vi "Dresden R2R Sputter 03.02.2018 IY24.vi"() -> ()   [LabVIEW 2009] (continued)
                    n2885 = stacked-sequence {
                      frame #0 {
                        n2886 = local write "Pps_code_entry"("PF174=" ("Pps_code_entry")) -> ()
                      }
                      frame #1 {
                        n2887 = Wait (ms)(milliseconds to wait=u32 500) -> ()  [unwired: 1 out]
                      }
                      frame #2 {
                        n2888 = local write "Ppsok"(TRUE ("Ppsok")) -> ()
                      }
                    }
                  }
                  frame #1 {
                    n2889 = stacked-sequence {
                      frame #0 {
                        n2890 = local write "Pps_code_entry"("PF173=" ("Pps_code_entry")) -> ()
                      }
                      frame #1 {
                        n2891 = Wait (ms)(milliseconds to wait=u32 500) -> ()  [unwired: 1 out]
                      }
                      frame #2 {
                        n2892 = local write "Ppsok"(TRUE ("Ppsok")) -> ()
                      }
                    }
                  }
                }
              }
            }
            n2893 = case shown="True" w4809 {
              tunnel: w4813 -> [_ w5102]
              frame #0 {
              }
              frame #1 {
                n2894 = case shown="False" w5102 {
                  frame #0 {
                    n2895 = stacked-sequence {
                      frame #0 {
                        n2896 = local write "Pps_code_entry"("PF206=" ("Pps_code_entry")) -> ()
                      }
                      frame #1 {
                        n2897 = Wait (ms)(milliseconds to wait=u32 500) -> ()  [unwired: 1 out]
                      }
                      frame #2 {
                        n2898 = local write "Ppsok"(TRUE ("Ppsok")) -> ()
                      }
                    }
                  }
                  frame #1 {
                    n2899 = stacked-sequence {
                      frame #0 {
                        n2900 = local write "Pps_code_entry"("PF205=" ("Pps_code_entry")) -> ()
                      }
                      frame #1 {
                        n2901 = Wait (ms)(milliseconds to wait=u32 500) -> ()  [unwired: 1 out]
                      }
                      frame #2 {
                        n2902 = local write "Ppsok"(TRUE ("Ppsok")) -> ()
                      }
                    }
                  }
                }
              }
            }
            n2903 = case shown="True" w4969 {
              tunnel: w4973 -> [_ w5333]
              frame #0 {
              }
              frame #1 {
                n2904 = case shown="False" w5333 {
                  frame #0 {
                    n2905 = stacked-sequence {
                      frame #0 {
                        n2906 = local write "Pps_code_entry"("PF138=" ("Pps_code_entry")) -> ()
                      }
                      frame #1 {
                        n2907 = Wait (ms)(milliseconds to wait=u32 500) -> ()  [unwired: 1 out]
                      }
                      frame #2 {
                        n2908 = local write "Ppsok"(TRUE ("Ppsok")) -> ()
                      }
                    }
                  }
                  frame #1 {
                    n2909 = stacked-sequence {
                      frame #0 {
                        n2910 = local write "Pps_code_entry"("PF137=" ("Pps_code_entry")) -> ()
                      }
                      frame #1 {
                        n2911 = Wait (ms)(milliseconds to wait=u32 500) -> ()  [unwired: 1 out]
                      }
                      frame #2 {
                        n2912 = local write "Ppsok"(TRUE ("Ppsok")) -> ()
                      }
                    }
                  }
                }
              }
            }
            n2913 = case shown="True" w4828 {
              tunnel: w4824 -> [_ w5081]
              frame #0 {
              }
              frame #1 {
                n2914 = case shown="False" w5081 {
                  frame #0 {
                    n2915 = stacked-sequence {
                      frame #0 {
                        n2916 = local write "Pps_code_entry"("PF208=" ("Pps_code_entry")) -> ()
                      }
                      frame #1 {
                        n2917 = Wait (ms)(milliseconds to wait=u32 500) -> ()  [unwired: 1 out]
                      }
                      frame #2 {
                        n2918 = local write "Ppsok"(TRUE ("Ppsok")) -> ()
                      }
                    }
                  }
                  frame #1 {
                    n2919 = stacked-sequence {
                      frame #0 {
                        n2920 = local write "Pps_code_entry"("PF207=" ("Pps_code_entry")) -> ()
                      }
                      frame #1 {
                        n2921 = Wait (ms)(milliseconds to wait=u32 500) -> ()  [unwired: 1 out]
                      }
                      frame #2 {
                        n2922 = local write "Ppsok"(TRUE ("Ppsok")) -> ()
                      }
                    }
                  }
                }
              }
            }
            n2923 = case shown="True" w4988 {
              tunnel: w4984 -> [_ w5312]
              frame #0 {
              }
              frame #1 {
                n2924 = case shown="False" w5312 {
                  frame #0 {
                    n2925 = stacked-sequence {
                      frame #0 {
                        n2926 = local write "Pps_code_entry"("PF140=" ("Pps_code_entry")) -> ()
                      }
                      frame #1 {
                        n2927 = Wait (ms)(milliseconds to wait=u32 500) -> ()  [unwired: 1 out]
                      }
                      frame #2 {
                        n2928 = local write "Ppsok"(TRUE ("Ppsok")) -> ()
                      }
                    }
                  }
                  frame #1 {
                    n2929 = stacked-sequence {
                      frame #0 {
                        n2930 = local write "Pps_code_entry"("PF139=" ("Pps_code_entry")) -> ()
                      }
                      frame #1 {
                        n2931 = Wait (ms)(milliseconds to wait=u32 500) -> ()  [unwired: 1 out]
                      }
                      frame #2 {
                        n2932 = local write "Ppsok"(TRUE ("Ppsok")) -> ()
                      }
                    }
                  }
                }
              }
            }
            n2933 = case shown="True" w4869 {
              tunnel: w4873 -> [_ w5235]
              frame #0 {
              }
              frame #1 {
                n2934 = case shown="False" w5235 {
                  frame #0 {
                    n2935 = stacked-sequence {
                      frame #0 {
                        n2936 = local write "Pps_code_entry"("PF170=" ("Pps_code_entry")) -> ()
                      }
                      frame #1 {
                        n2937 = Wait (ms)(milliseconds to wait=u32 500) -> ()  [unwired: 1 out]
                      }
                      frame #2 {
                        n2938 = local write "Ppsok"(TRUE ("Ppsok")) -> ()
                      }
                    }
                  }
                  frame #1 {
                    n2939 = stacked-sequence {
                      frame #0 {
                        n2940 = local write "Pps_code_entry"("PF169=" ("Pps_code_entry")) -> ()
                      }
                      frame #1 {
                        n2941 = Wait (ms)(milliseconds to wait=u32 500) -> ()  [unwired: 1 out]
                      }
                      frame #2 {
                        n2942 = local write "Ppsok"(TRUE ("Ppsok")) -> ()
                      }
                    }
                  }
                }
              }
            }
            n2943 = case shown="True" w4904 {
              tunnel: w4908 -> [_ w5179]
              frame #0 {
              }
              frame #1 {
                n2944 = case shown="False" w5179 {
                  frame #0 {
                    n2945 = stacked-sequence {
                      frame #0 {
                        n2946 = local write "Pps_code_entry"("PF184=" ("Pps_code_entry")) -> ()
                      }
                      frame #1 {
                        n2947 = Wait (ms)(milliseconds to wait=u32 500) -> ()  [unwired: 1 out]
                      }
                      frame #2 {
                        n2948 = local write "Ppsok"(TRUE ("Ppsok")) -> ()
                      }
                    }
                  }
                  frame #1 {
                    n2949 = stacked-sequence {
                      frame #0 {
                        n2950 = local write "Pps_code_entry"("PF183=" ("Pps_code_entry")) -> ()
                      }
                      frame #1 {
                        n2951 = Wait (ms)(milliseconds to wait=u32 500) -> ()  [unwired: 1 out]
                      }
                      frame #2 {
                        n2952 = local write "Ppsok"(TRUE ("Ppsok")) -> ()
                      }
                    }
                  }
                }
              }
            }
            n2953 = case shown="True" w4798 {
              tunnel: w4794 -> [_ w5123]
              frame #0 {
              }
              frame #1 {
                n2954 = case shown="True" w5123 {
                  frame #0 {
                    n2955 = stacked-sequence {
                      frame #0 {
                        n2956 = local write "Pps_code_entry"("PF204=" ("Pps_code_entry")) -> ()
                      }
                      frame #1 {
                        n2957 = Wait (ms)(milliseconds to wait=u32 500) -> ()  [unwired: 1 out]
                      }
                      frame #2 {
                        n2958 = local write "Ppsok"(TRUE ("Ppsok")) -> ()
                      }
                    }
                  }
                  frame #1 {
                    n2959 = stacked-sequence {
                      frame #0 {
                        n2960 = local write "Pps_code_entry"("PF203=" ("Pps_code_entry")) -> ()
                      }
                      frame #1 {
                        n2961 = Wait (ms)(milliseconds to wait=u32 500) -> ()  [unwired: 1 out]
                      }
                      frame #2 {
                        n2962 = local write "Ppsok"(TRUE ("Ppsok")) -> ()
                      }
                    }
                  }
                }
              }
            }
            n2963 = case shown="True" w5028 {
              tunnel: w5024 -> [_ w5438]
              frame #0 {
              }
              frame #1 {
                n2964 = case shown="True" w5438 {
                  frame #0 {
                    n2965 = stacked-sequence {
                      frame #0 {
                        n2966 = local write "Pps_code_entry"("PF108=" ("Pps_code_entry")) -> ()
                      }
                      frame #1 {
                        n2967 = Wait (ms)(milliseconds to wait=u32 500) -> ()  [unwired: 1 out]
                      }
                      frame #2 {
                        n2968 = local write "Ppsok"(TRUE ("Ppsok")) -> ()
                      }
                    }
                  }
                  frame #1 {
                    n2969 = stacked-sequence {
                      frame #0 {
                        n2970 = local write "Pps_code_entry"("PF107=" ("Pps_code_entry")) -> ()
                      }
                      frame #1 {
                        n2971 = Wait (ms)(milliseconds to wait=u32 500) -> ()  [unwired: 1 out]
                      }
                      frame #2 {
                        n2972 = local write "Ppsok"(TRUE ("Ppsok")) -> ()
                      }
                    }
                  }
                }
              }
            }
            n2973 = case shown="True" w4958 {
              tunnel: w4954 -> [_ w5354]
              frame #0 {
              }
              frame #1 {
                n2974 = case shown="True" w5354 {
                  frame #0 {
                    n2975 = stacked-sequence {
                      frame #0 {
                        n2976 = local write "Pps_code_entry"("PF136=" ("Pps_code_entry")) -> ()
                      }
                      frame #1 {
                        n2977 = Wait (ms)(milliseconds to wait=u32 500) -> ()  [unwired: 1 out]
                      }
                      frame #2 {
                        n2978 = local write "Ppsok"(TRUE ("Ppsok")) -> ()
                      }
                    }
                  }
                  frame #1 {
                    n2979 = stacked-sequence {
                      frame #0 {
                        n2980 = local write "Pps_code_entry"("PF135=" ("Pps_code_entry")) -> ()
                      }
                      frame #1 {
                        n2981 = Wait (ms)(milliseconds to wait=u32 500) -> ()  [unwired: 1 out]
                      }
                      frame #2 {
                        n2982 = local write "Ppsok"(TRUE ("Ppsok")) -> ()
                      }
                    }
                  }
                }
              }
            }
            n2983 = case shown="True" w4923 {
              tunnel: w4919 -> [_ w5291]
              frame #0 {
              }
              frame #1 {
                n2984 = case shown="True" w5291 {
                  frame #0 {
                    n2985 = stacked-sequence {
                      frame #0 {
                        n2986 = local write "Pps_code_entry"("PF150=" ("Pps_code_entry")) -> ()
                      }
                      frame #1 {
                        n2987 = Wait (ms)(milliseconds to wait=u32 500) -> ()  [unwired: 1 out]
                      }
                      frame #2 {
                        n2988 = local write "Ppsok"(TRUE ("Ppsok")) -> ()
                      }
                    }
                  }
                  frame #1 {
                    n2989 = stacked-sequence {
                      frame #0 {
                        n2990 = local write "Pps_code_entry"("PF149=" ("Pps_code_entry")) -> ()
                      }
                      frame #1 {
                        n2991 = Wait (ms)(milliseconds to wait=u32 500) -> ()  [unwired: 1 out]
                      }
                      frame #2 {
                        n2992 = local write "Ppsok"(TRUE ("Ppsok")) -> ()
                      }
                    }
                  }
                }
              }
            }
            n2993 = case shown="True" w5009 {
              tunnel: w5013 -> [_ w5417]
              frame #0 {
              }
              frame #1 {
                n2994 = case shown="False" w5417 {
                  frame #0 {
                    n2995 = stacked-sequence {
                      frame #0 {
                        n2996 = local write "Pps_code_entry"("PF110=" ("Pps_code_entry")) -> ()
                      }
                      frame #1 {
                        n2997 = Wait (ms)(milliseconds to wait=u32 500) -> ()  [unwired: 1 out]
                      }
                      frame #2 {
                        n2998 = local write "Ppsok"(TRUE ("Ppsok")) -> ()
                      }
                    }
                  }
                  frame #1 {
                    n2999 = stacked-sequence {
                      frame #0 {
                        n3000 = local write "Pps_code_entry"("PF109=" ("Pps_code_entry")) -> ()
                      }
                      frame #1 {
                        n3001 = Wait (ms)(milliseconds to wait=u32 500) -> ()  [unwired: 1 out]
                      }
                      frame #2 {
                        n3002 = local write "Ppsok"(TRUE ("Ppsok")) -> ()
                      }
                    }
                  }
                }
              }
            }
            n3003 = case shown="True" w4900 {
              tunnel: w4899 -> [_ w5277]
              frame #0 {
              }
              frame #1 {
                n3004 = case shown="False" w5277 {
                  frame #0 {
                    n3005 = stacked-sequence {
                      frame #0 {
                        n3006 = local write "Pps_code_entry"("PF166=" ("Pps_code_entry")) -> ()
                      }
                      frame #1 {
                        n3007 = Wait (ms)(milliseconds to wait=u32 500) -> ()  [unwired: 1 out]
                      }
                      frame #2 {
                        n3008 = local write "Ppsok"(TRUE ("Ppsok")) -> ()
                      }
                    }
                  }
                  frame #1 {
                    n3009 = stacked-sequence {
                      frame #0 {
                        n3010 = local write "Pps_code_entry"("PF165=" ("Pps_code_entry")) -> ()
                      }
                      frame #1 {
                        n3011 = Wait (ms)(milliseconds to wait=u32 500) -> ()  [unwired: 1 out]
                      }
                      frame #2 {
                        n3012 = local write "Ppsok"(TRUE ("Ppsok")) -> ()
                      }
                    }
                  }
                }
              }
            }
            n3013 = case shown="True" w4898 {
              tunnel: w4894 -> [_ w5270]
              frame #0 {
              }
              frame #1 {
                n3014 = case shown="False" w5270 {
                  frame #0 {
                    n3015 = stacked-sequence {
                      frame #0 {
                        n3016 = local write "Pps_code_entry"("PF168=" ("Pps_code_entry")) -> ()
                      }
                      frame #1 {
                        n3017 = Wait (ms)(milliseconds to wait=u32 500) -> ()  [unwired: 1 out]
                      }
                      frame #2 {
                        n3018 = local write "Ppsok"(TRUE ("Ppsok")) -> ()
                      }
                    }
                  }
                  frame #1 {
                    n3019 = stacked-sequence {
                      frame #0 {
                        n3020 = local write "Pps_code_entry"("PF167=" ("Pps_code_entry")) -> ()
                      }
                      frame #1 {
                        n3021 = Wait (ms)(milliseconds to wait=u32 500) -> ()  [unwired: 1 out]
                      }
                      frame #2 {
                        n3022 = local write "Ppsok"(TRUE ("Ppsok")) -> ()
                      }
                    }
                  }
                }
              }
            }
            n3023 = case shown="True" w5039 {
              tunnel: w5043 -> [_ w5459]
              frame #0 {
              }
              frame #1 {
                n3024 = case shown="False" w5459 {
                  frame #0 {
                    n3025 = stacked-sequence {
                      frame #0 {
                        n3026 = local write "Pps_code_entry"("PF106=" ("Pps_code_entry")) -> ()
                      }
                      frame #1 {
                        n3027 = Wait (ms)(milliseconds to wait=u32 500) -> ()  [unwired: 1 out]
                      }
                      frame #2 {
                        n3028 = local write "Ppsok"(TRUE ("Ppsok")) -> ()
                      }
                    }
                  }
                  frame #1 {
                    n3029 = stacked-sequence {
                      frame #0 {
                        n3030 = local write "Pps_code_entry"("PF105=" ("Pps_code_entry")) -> ()
                      }
                      frame #1 {
                        n3031 = Wait (ms)(milliseconds to wait=u32 500) -> ()  [unwired: 1 out]
                      }
                      frame #2 {
                        n3032 = local write "Ppsok"(TRUE ("Ppsok")) -> ()
                      }
                    }
                  }
                }
              }
            }
            n3033 = case shown="True" w4767 {
              tunnel: w4768 -> [_ w5165]
              frame #0 {
              }
              frame #1 {
                n3034 = case shown="True" w5165 {
                  frame #0 {
                    n3035 = stacked-sequence {
                      frame #0 {
                        n3036 = local write "Pps_code_entry"("PF200=" ("Pps_code_entry")) -> ()
                      }
                      frame #1 {
                        n3037 = Wait (ms)(milliseconds to wait=u32 500) -> ()  [unwired: 1 out]
                      }
                      frame #2 {
                        n3038 = local write "Ppsok"(TRUE ("Ppsok")) -> ()
                      }
                    }
                  }
                  frame #1 {
                    n3039 = stacked-sequence {
                      frame #0 {
                        n3040 = local write "Pps_code_entry"("PF199=" ("Pps_code_entry")) -> ()
                      }
                      frame #1 {
                        n3041 = Wait (ms)(milliseconds to wait=u32 500) -> ()  [unwired: 1 out]
                      }
                      frame #2 {
                        n3042 = local write "Ppsok"(TRUE ("Ppsok")) -> ()
                      }
                    }
                  }
                }
              }
            }
            n3043 = case shown="True" w4769 {
              tunnel: w4773 -> [_ w5158]
              frame #0 {
              }
              frame #1 {
                n3044 = case shown="True" w5158 {
                  frame #0 {
                    n3045 = stacked-sequence {
                      frame #0 {
                        n3046 = local write "Pps_code_entry"("PF202=" ("Pps_code_entry")) -> ()
                      }
                      frame #1 {
                        n3047 = Wait (ms)(milliseconds to wait=u32 500) -> ()  [unwired: 1 out]
                      }
                      frame #2 {
                        n3048 = local write "Ppsok"(TRUE ("Ppsok")) -> ()
                      }
                    }
                  }
                  frame #1 {
                    n3049 = stacked-sequence {
                      frame #0 {
                        n3050 = local write "Pps_code_entry"("PF201=" ("Pps_code_entry")) -> ()
                      }
                      frame #1 {
                        n3051 = Wait (ms)(milliseconds to wait=u32 500) -> ()  [unwired: 1 out]
                      }
                      frame #2 {
                        n3052 = local write "Ppsok"(TRUE ("Ppsok")) -> ()
                      }
                    }
                  }
                }
              }
            }
            n3053 = case shown="True" w4927 {
              tunnel: w4928 -> [_ w5396]
              frame #0 {
              }
              frame #1 {
                n3054 = case shown="False" w5396 {
                  frame #0 {
                    n3055 = stacked-sequence {
                      frame #0 {
                        n3056 = local write "Pps_code_entry"("PF133=" ("Pps_code_entry")) -> ()
                      }
                      frame #1 {
                        n3057 = Wait (ms)(milliseconds to wait=u32 500) -> ()  [unwired: 1 out]
                      }
                      frame #2 {
                        n3058 = local write "Ppsok"(TRUE ("Ppsok")) -> ()
                      }
                    }
                  }
                  frame #1 {
                    n3059 = stacked-sequence {
                      frame #0 {
                        n3060 = local write "Pps_code_entry"("PF131=" ("Pps_code_entry")) -> ()
                      }
                      frame #1 {
                        n3061 = Wait (ms)(milliseconds to wait=u32 500) -> ()  [unwired: 1 out]
                      }
                      frame #2 {
                        n3062 = local write "Ppsok"(TRUE ("Ppsok")) -> ()
                      }
                    }
                  }
                }
              }
            }
            n3063 = case shown="True" w4929 {
              tunnel: w4933 -> [_ w5389]
              frame #0 {
              }
              frame #1 {
                n3064 = case shown="True" w5389 {
                  frame #0 {
                    n3065 = stacked-sequence {
                      frame #0 {
                        n3066 = local write "Pps_code_entry"("PF134=" ("Pps_code_entry")) -> ()
                      }
                      frame #1 {
                        n3067 = Wait (ms)(milliseconds to wait=u32 500) -> ()  [unwired: 1 out]
                      }
                      frame #2 {
                        n3068 = local write "Ppsok"(TRUE ("Ppsok")) -> ()
                      }
                    }
                  }
                  frame #1 {
                    n3069 = stacked-sequence {
                      frame #0 {
                        n3070 = local write "Pps_code_entry"("PF133=" ("Pps_code_entry")) -> ()
                      }
                      frame #1 {
                        n3071 = Wait (ms)(milliseconds to wait=u32 500) -> ()  [unwired: 1 out]
                      }
                      frame #2 {
                        n3072 = local write "Ppsok"(TRUE ("Ppsok")) -> ()
                      }
                    }
                  }
                }
              }
            }
            n3073 = case shown="True" w5070 {
              tunnel: w5069 -> [_ w5501]
              frame #0 {
              }
              frame #1 {
                n3074 = case shown="True" w5501 {
                  frame #0 {
                    n3075 = stacked-sequence {
                      frame #0 {
                        n3076 = local write "Pps_code_entry"("PF102=" ("Pps_code_entry")) -> ()
                      }
                      frame #1 {
                        n3077 = Wait (ms)(milliseconds to wait=u32 500) -> ()  [unwired: 1 out]
                      }
                      frame #2 {
                        n3078 = local write "Ppsok"(TRUE ("Ppsok")) -> ()
                      }
                    }
                  }
                  frame #1 {
                    n3079 = stacked-sequence {
                      frame #0 {
                        n3080 = local write "Pps_code_entry"("PF101=" ("Pps_code_entry")) -> ()
                      }
                      frame #1 {
                        n3081 = Wait (ms)(milliseconds to wait=u32 500) -> ()  [unwired: 1 out]
                      }
                      frame #2 {
                        n3082 = local write "Ppsok"(TRUE ("Ppsok")) -> ()
                      }
                    }
                  }
                }
              }
            }
            n3083 = case shown="True" w5068 {
              tunnel: w5064 -> [_ w5494]
              frame #0 {
              }
              frame #1 {
                n3084 = case shown="False" w5494 {
                  frame #0 {
                    n3085 = stacked-sequence {
                      frame #0 {
                        n3086 = local write "Pps_code_entry"("PF104=" ("Pps_code_entry")) -> ()
                      }
                      frame #1 {
                        n3087 = Wait (ms)(milliseconds to wait=u32 500) -> ()  [unwired: 1 out]
                      }
                      frame #2 {
                        n3088 = local write "Ppsok"(TRUE ("Ppsok")) -> ()
                      }
                    }
                  }
                  frame #1 {
                    n3089 = stacked-sequence {
                      frame #0 {
                        n3090 = local write "Pps_code_entry"("PF103=" ("Pps_code_entry")) -> ()
                      }
                      frame #1 {
                        n3091 = Wait (ms)(milliseconds to wait=u32 500) -> ()  [unwired: 1 out]
                      }
                      frame #2 {
                        n3092 = local write "Ppsok"(TRUE ("Ppsok")) -> ()
                      }
                    }
                  }
                }
              }
            }
            n3093 = local read "Ch3_Trns_gv_bp2_on"() -> (w4853:bool)
            n3094 = local read "Ch2_Trns_gv_bp2_on"() -> (w4974:bool)
            n3095 = local read "Ch4_Trns_gv_bp_on"() -> (w4814:bool)
            n3096 = local read "Ch1_Trns_gv_bp2_on"() -> (w5023:bool)
            n3097 = local read "Ch3_Trns_gv_bp_on"() -> (w4909:bool)
            n3098 = local read "Ch2_Trns_gv_bp_on"() -> (w4918:bool)
            n3099 = local read "Ch3_Bp_bv_on_R"() -> (w4864:bool)
            n3100 = local read "Ch4_Bp_bv_on_L"() -> (w4803:bool)
            n3101 = local read "Ch2_Bp_bv_on_R"() -> (w4963:bool)
            n3102 = local read "Ch3_Pc_bv_on"() -> (w4834:bool)
            n3103 = local read "Ch4_Pc_bv_on"() -> (w4833:bool)
            n3104 = local read "Ch2_Pc_bv_on"() -> (w4993:bool)
            n3105 = local read "Ch1_Bp_bv_on_R"() -> (w5034:bool)
            n3106 = local read "Ch3_Tp_bv_on"() -> (w4884:bool)
            n3107 = local read "Ch4_Tp_bv_on"() -> (w4783:bool)
            n3108 = local read "Ch1_Pc_bv_on"() -> (w5004:bool)
            n3109 = local read "Ch2_Tp_bv_on"() -> (w4943:bool)
            n3110 = local read "Ch3_Tp_on"() -> (w4893:bool)
            n3111 = local read "Ch4_Tp_on"() -> (w4774:bool)
            n3112 = local read "Ch1_Tp_bv_on"() -> (w5054:bool)
            n3113 = local read "Ch2_Tp_on"() -> (w4934:bool)
            n3114 = local read "Ch1_Tp_on"() -> (w5063:bool)
            n3115 = feedback #76() -> (w4852:bool)  [unwired: 1 in]
            n3116 = feedback #77() -> (w4892:bool)  [unwired: 1 in]
            n3117 = feedback #78() -> (w4815:bool)  [unwired: 1 in]
            n3118 = feedback #79() -> (w4975:bool)  [unwired: 1 in]
            n3119 = feedback #80() -> (w4775:bool)  [unwired: 1 in]
            n3120 = feedback #81() -> (w4935:bool)  [unwired: 1 in]
            n3121 = feedback #82() -> (w4835:bool)  [unwired: 1 in]
            n3122 = feedback #83() -> (w5022:bool)  [unwired: 1 in]
            n3123 = feedback #84() -> (w4832:bool)  [unwired: 1 in]
            n3124 = feedback #85() -> (w5062:bool)  [unwired: 1 in]
            n3125 = feedback #86() -> (w4992:bool)  [unwired: 1 in]
            n3126 = feedback #87() -> (w4885:bool)  [unwired: 1 in]
            n3127 = feedback #88() -> (w4910:bool)  [unwired: 1 in]
            n3128 = feedback #89() -> (w4865:bool)  [unwired: 1 in]
            n3129 = feedback #90() -> (w4782:bool)  [unwired: 1 in]
            n3130 = feedback #91() -> (w5005:bool)  [unwired: 1 in]
            n3131 = feedback #92() -> (w4942:bool)  [unwired: 1 in]
            n3132 = feedback #93() -> (w4917:bool)  [unwired: 1 in]
            n3133 = feedback #94() -> (w4802:bool)  [unwired: 1 in]
            n3134 = feedback #95() -> (w4962:bool)  [unwired: 1 in]
            n3135 = feedback #96() -> (w5055:bool)  [unwired: 1 in]
            n3136 = feedback #97() -> (w5035:bool)  [unwired: 1 in]
            n3137 = Boolean To (0,1)(Boolean=w4853) -> (0, 1=w4851:i16)
            n3138 = Boolean To (0,1)(Boolean=w4852) -> (0, 1=w4850:i16)
            n3139 = Boolean To (0,1)(Boolean=w4893) -> (0, 1=w4891:i16)
            n3140 = Boolean To (0,1)(Boolean=w4892) -> (0, 1=w4890:i16)
            n3141 = Boolean To (0,1)(Boolean=w4814) -> (0, 1=w4816:i16)
            n3142 = Boolean To (0,1)(Boolean=w4815) -> (0, 1=w4817:i16)
            n3143 = Boolean To (0,1)(Boolean=w4974) -> (0, 1=w4976:i16)
            n3144 = Boolean To (0,1)(Boolean=w4975) -> (0, 1=w4977:i16)
            n3145 = Boolean To (0,1)(Boolean=w4774) -> (0, 1=w4776:i16)
            n3146 = Boolean To (0,1)(Boolean=w4775) -> (0, 1=w4777:i16)
            n3147 = Boolean To (0,1)(Boolean=w4934) -> (0, 1=w4936:i16)
            n3148 = Boolean To (0,1)(Boolean=w4935) -> (0, 1=w4937:i16)
            n3149 = Boolean To (0,1)(Boolean=w4834) -> (0, 1=w4836:i16)
            n3150 = Boolean To (0,1)(Boolean=w4835) -> (0, 1=w4837:i16)
            n3151 = Boolean To (0,1)(Boolean=w5023) -> (0, 1=w5021:i16)
            n3152 = Boolean To (0,1)(Boolean=w5022) -> (0, 1=w5020:i16)
            n3153 = Boolean To (0,1)(Boolean=w4833) -> (0, 1=w4831:i16)
            n3154 = Boolean To (0,1)(Boolean=w4832) -> (0, 1=w4830:i16)
            n3155 = Boolean To (0,1)(Boolean=w5063) -> (0, 1=w5061:i16)
            n3156 = Boolean To (0,1)(Boolean=w5062) -> (0, 1=w5060:i16)
            n3157 = Boolean To (0,1)(Boolean=w4993) -> (0, 1=w4991:i16)
            n3158 = Boolean To (0,1)(Boolean=w4992) -> (0, 1=w4990:i16)
            n3159 = Boolean To (0,1)(Boolean=w4884) -> (0, 1=w4886:i16)
            n3160 = Boolean To (0,1)(Boolean=w4885) -> (0, 1=w4887:i16)
            n3161 = Boolean To (0,1)(Boolean=w4909) -> (0, 1=w4911:i16)
            n3162 = Boolean To (0,1)(Boolean=w4910) -> (0, 1=w4912:i16)
            n3163 = Boolean To (0,1)(Boolean=w4864) -> (0, 1=w4866:i16)
            n3164 = Boolean To (0,1)(Boolean=w4865) -> (0, 1=w4867:i16)
            n3165 = Boolean To (0,1)(Boolean=w4783) -> (0, 1=w4781:i16)
            n3166 = Boolean To (0,1)(Boolean=w4782) -> (0, 1=w4780:i16)
            n3167 = Boolean To (0,1)(Boolean=w5004) -> (0, 1=w5006:i16)
            n3168 = Boolean To (0,1)(Boolean=w5005) -> (0, 1=w5007:i16)
            n3169 = Boolean To (0,1)(Boolean=w4943) -> (0, 1=w4941:i16)
            n3170 = Boolean To (0,1)(Boolean=w4942) -> (0, 1=w4940:i16)
            n3171 = Boolean To (0,1)(Boolean=w4918) -> (0, 1=w4916:i16)
            n3172 = Boolean To (0,1)(Boolean=w4917) -> (0, 1=w4915:i16)
            n3173 = Boolean To (0,1)(Boolean=w4803) -> (0, 1=w4801:i16)
            n3174 = Boolean To (0,1)(Boolean=w4802) -> (0, 1=w4800:i16)
            n3175 = Boolean To (0,1)(Boolean=w4963) -> (0, 1=w4961:i16)
            n3176 = Boolean To (0,1)(Boolean=w4962) -> (0, 1=w4960:i16)
            n3177 = Boolean To (0,1)(Boolean=w5054) -> (0, 1=w5056:i16)
            n3178 = Boolean To (0,1)(Boolean=w5055) -> (0, 1=w5057:i16)
            n3179 = Boolean To (0,1)(Boolean=w5034) -> (0, 1=w5036:i16)
            n3180 = Boolean To (0,1)(Boolean=w5035) -> (0, 1=w5037:i16)
            n3181 = Not Equal?(x=w4851, y=w4850) -> (x != y?=w4849:bool)
            n3182 = Not Equal?(x=w4891, y=w4890) -> (x != y?=w4889:bool)
            n3183 = Not Equal?(x=w4816, y=w4817) -> (x != y?=w4818:bool)
            n3184 = Not Equal?(x=w4976, y=w4977) -> (x != y?=w4978:bool)
            n3185 = Not Equal?(x=w4776, y=w4777) -> (x != y?=w4778:bool)
            n3186 = Not Equal?(x=w4936, y=w4937) -> (x != y?=w4938:bool)
            n3187 = Not Equal?(x=w4836, y=w4837) -> (x != y?=w4838:bool)
            n3188 = Not Equal?(x=w5021, y=w5020) -> (x != y?=w5019:bool)
            n3189 = Not Equal?(x=w4831, y=w4830) -> (x != y?=w4829:bool)
            n3190 = Not Equal?(x=w5061, y=w5060) -> (x != y?=w5059:bool)
            n3191 = Not Equal?(x=w4991, y=w4990) -> (x != y?=w4989:bool)
            n3192 = Not Equal?(x=w4886, y=w4887) -> (x != y?=w4888:bool)
            n3193 = Not Equal?(x=w4911, y=w4912) -> (x != y?=w4913:bool)
            n3194 = Not Equal?(x=w4866, y=w4867) -> (x != y?=w4868:bool)
            n3195 = Not Equal?(x=w4781, y=w4780) -> (x != y?=w4779:bool)
            n3196 = Not Equal?(x=w5006, y=w5007) -> (x != y?=w5008:bool)
            n3197 = Not Equal?(x=w4941, y=w4940) -> (x != y?=w4939:bool)
            n3198 = Not Equal?(x=w4916, y=w4915) -> (x != y?=w4914:bool)
            n3199 = Not Equal?(x=w4801, y=w4800) -> (x != y?=w4799:bool)
            n3200 = Not Equal?(x=w4961, y=w4960) -> (x != y?=w4959:bool)
            n3201 = Not Equal?(x=w5056, y=w5057) -> (x != y?=w5058:bool)
            n3202 = Not Equal?(x=w5036, y=w5037) -> (x != y?=w5038:bool)
            n3203 = case shown="True" w4849 {
              tunnel: w4853 -> [_ w5207]
              frame #0 {
              }
              frame #1 {
                n3204 = case shown="False" w5207 {
                  frame #0 {
                    n3205 = stacked-sequence {
                      frame #0 {
                        n3206 = local write "Pps_code_entry"("PF182=" ("Pps_code_entry")) -> ()
                      }
                      frame #1 {
                        n3207 = Wait (ms)(milliseconds to wait=u32 500) -> ()  [unwired: 1 out]
                      }
                      frame #2 {
                        n3208 = local write "Ppsok"(TRUE ("Ppsok")) -> ()
                      }
                    }
                  }
                  frame #1 {
                    n3209 = stacked-sequence {
                      frame #0 {
                        n3210 = local write "Pps_code_entry"("PF181=" ("Pps_code_entry")) -> ()
                      }
                      frame #1 {
                        n3211 = Wait (ms)(milliseconds to wait=u32 500) -> ()  [unwired: 1 out]
                      }
                      frame #2 {
                        n3212 = local write "Ppsok"(TRUE ("Ppsok")) -> ()
                      }
                    }
                  }
                }
              }
            }
            n3213 = case shown="True" w4889 {
              tunnel: w4893 -> [_ w5263]
              frame #0 {
              }
              frame #1 {
                n3214 = case shown="True" w5263 {
                  frame #0 {
                    n3215 = stacked-sequence {
                      frame #0 {
                        n3216 = local write "Pps_code_entry"("PF178=" ("Pps_code_entry")) -> ()
                      }
                      frame #1 {
                        n3217 = Wait (ms)(milliseconds to wait=u32 500) -> ()  [unwired: 1 out]
                      }
                      frame #2 {
                        n3218 = local write "Ppsok"(TRUE ("Ppsok")) -> ()
                      }
                    }
                  }
                  frame #1 {
                    n3219 = stacked-sequence {
                      frame #0 {
                        n3220 = local write "Pps_code_entry"("PF177=" ("Pps_code_entry")) -> ()
                      }
                      frame #1 {
                        n3221 = Wait (ms)(milliseconds to wait=u32 500) -> ()  [unwired: 1 out]
                      }
                      frame #2 {
                        n3222 = local write "Ppsok"(TRUE ("Ppsok")) -> ()
                      }
                    }
                  }
                }
              }
            }
            n3223 = case shown="True" w4818 {
              tunnel: w4814 -> [_ w5095]
              frame #0 {
              }
              frame #1 {
                n3224 = case shown="True" w5095 {
                  frame #0 {
                    n3225 = stacked-sequence {
                      frame #0 {
                        n3226 = local write "Pps_code_entry"("PF216=" ("Pps_code_entry")) -> ()
                      }
                      frame #1 {
                        n3227 = Wait (ms)(milliseconds to wait=u32 500) -> ()  [unwired: 1 out]
                      }
                      frame #2 {
                        n3228 = local write "Ppsok"(TRUE ("Ppsok")) -> ()
                      }
                    }
                  }
                  frame #1 {
                    n3229 = stacked-sequence {
                      frame #0 {
                        n3230 = local write "Pps_code_entry"("PF215=" ("Pps_code_entry")) -> ()
                      }
                      frame #1 {
                        n3231 = Wait (ms)(milliseconds to wait=u32 500) -> ()  [unwired: 1 out]
                      }
                      frame #2 {
                        n3232 = local write "Ppsok"(TRUE ("Ppsok")) -> ()
                      }
                    }
                  }
                }
              }
            }
            n3233 = case shown="True" w4978 {
              tunnel: w4974 -> [_ w5326]
              frame #0 {
              }
              frame #1 {
                n3234 = case shown="False" w5326 {
                  frame #0 {
                    n3235 = stacked-sequence {
                      frame #0 {
                        n3236 = local write "Pps_code_entry"("PF148=" ("Pps_code_entry")) -> ()
                      }
                      frame #1 {
                        n3237 = Wait (ms)(milliseconds to wait=u32 500) -> ()  [unwired: 1 out]
                      }
                      frame #2 {
                        n3238 = local write "Ppsok"(TRUE ("Ppsok")) -> ()
                      }
                    }
                  }
                  frame #1 {
                    n3239 = stacked-sequence {
                      frame #0 {
                        n3240 = local write "Pps_code_entry"("PF147=" ("Pps_code_entry")) -> ()
                      }
                      frame #1 {
                        n3241 = Wait (ms)(milliseconds to wait=u32 500) -> ()  [unwired: 1 out]
                      }
                      frame #2 {
                        n3242 = local write "Ppsok"(TRUE ("Ppsok")) -> ()
                      }
                    }
                  }
                }
              }
            }
            n3243 = case shown="True" w4778 {
              tunnel: w4774 -> [_ w5151]
              frame #0 {
              }
              frame #1 {
                n3244 = case shown="True" w5151 {
                  frame #0 {
                    n3245 = stacked-sequence {
                      frame #0 {
                        n3246 = local write "Pps_code_entry"("PF212=" ("Pps_code_entry")) -> ()
                      }
                      frame #1 {
                        n3247 = Wait (ms)(milliseconds to wait=u32 500) -> ()  [unwired: 1 out]
                      }
                      frame #2 {
                        n3248 = local write "Ppsok"(TRUE ("Ppsok")) -> ()
                      }
                    }
                  }
                  frame #1 {
                    n3249 = stacked-sequence {
                      frame #0 {
                        n3250 = local write "Pps_code_entry"("PF211=" ("Pps_code_entry")) -> ()
                      }
                      frame #1 {
                        n3251 = Wait (ms)(milliseconds to wait=u32 500) -> ()  [unwired: 1 out]
                      }
                      frame #2 {
                        n3252 = local write "Ppsok"(TRUE ("Ppsok")) -> ()
                      }
                    }
                  }
                }
              }
            }
            n3253 = case shown="True" w4938 {
              tunnel: w4934 -> [_ w5382]
              frame #0 {
              }
              frame #1 {
                n3254 = case shown="True" w5382 {
                  frame #0 {
                    n3255 = stacked-sequence {
                      frame #0 {
                        n3256 = local write "Pps_code_entry"("PF144=" ("Pps_code_entry")) -> ()
                      }
                      frame #1 {
                        n3257 = Wait (ms)(milliseconds to wait=u32 500) -> ()  [unwired: 1 out]
                      }
                      frame #2 {
                        n3258 = local write "Ppsok"(TRUE ("Ppsok")) -> ()
                      }
                    }
                  }
                  frame #1 {
                    n3259 = stacked-sequence {
                      frame #0 {
                        n3260 = local write "Pps_code_entry"("PF143=" ("Pps_code_entry")) -> ()
                      }
                      frame #1 {
                        n3261 = Wait (ms)(milliseconds to wait=u32 500) -> ()  [unwired: 1 out]
                      }
                      frame #2 {
                        n3262 = local write "Ppsok"(TRUE ("Ppsok")) -> ()
                      }
                    }
                  }
                }
              }
            }
            n3263 = case shown="True" w4838 {
              tunnel: w4834 -> [_ w5186]
              frame #0 {
              }
              frame #1 {
                n3264 = case shown="False" w5186 {
                  frame #0 {
                    n3265 = stacked-sequence {
                      frame #0 {
                        n3266 = local write "Pps_code_entry"("PF188=" ("Pps_code_entry")) -> ()
                      }
                      frame #1 {
                        n3267 = Wait (ms)(milliseconds to wait=u32 500) -> ()  [unwired: 1 out]
                      }
                      frame #2 {
                        n3268 = local write "Ppsok"(TRUE ("Ppsok")) -> ()
                      }
                    }
                  }
                  frame #1 {
                    n3269 = stacked-sequence {
                      frame #0 {